vi "Planta pilot.vi"() -> ()   [LabVIEW 2022 SP3]
panel:
  out "Numeric 6":dbl
  out "Numeric 5":dbl
  out "Numeric 4":dbl
  out "Numeric 3":dbl
  out "Numeric 2":dbl
  out "Boolean":bool
  out "Numeric":dbl
  out "Presión tanque alta":dbl[](graph)
  out "Presión tanque baja":dbl[](graph)
  out "Producción de Hidrogeno":dbl[](graph)
  out "Producción Solar":dbl[](graph)
  in  "stop":bool
  # "H2"
  # "H2 baja presión"
  # "H2 alta presión"
  # "Tanc baixa pressió"
  # "barg"
  # "Tanc alta pressió"
  # "Electrolizador"
  # "Compresor"
  # "kg/h"
  # "barg"
  # "Solar"
  # "Fuel Cell"
  # "kW"
  # "kg"
  # "kW"
  # "Xarxa electrica"
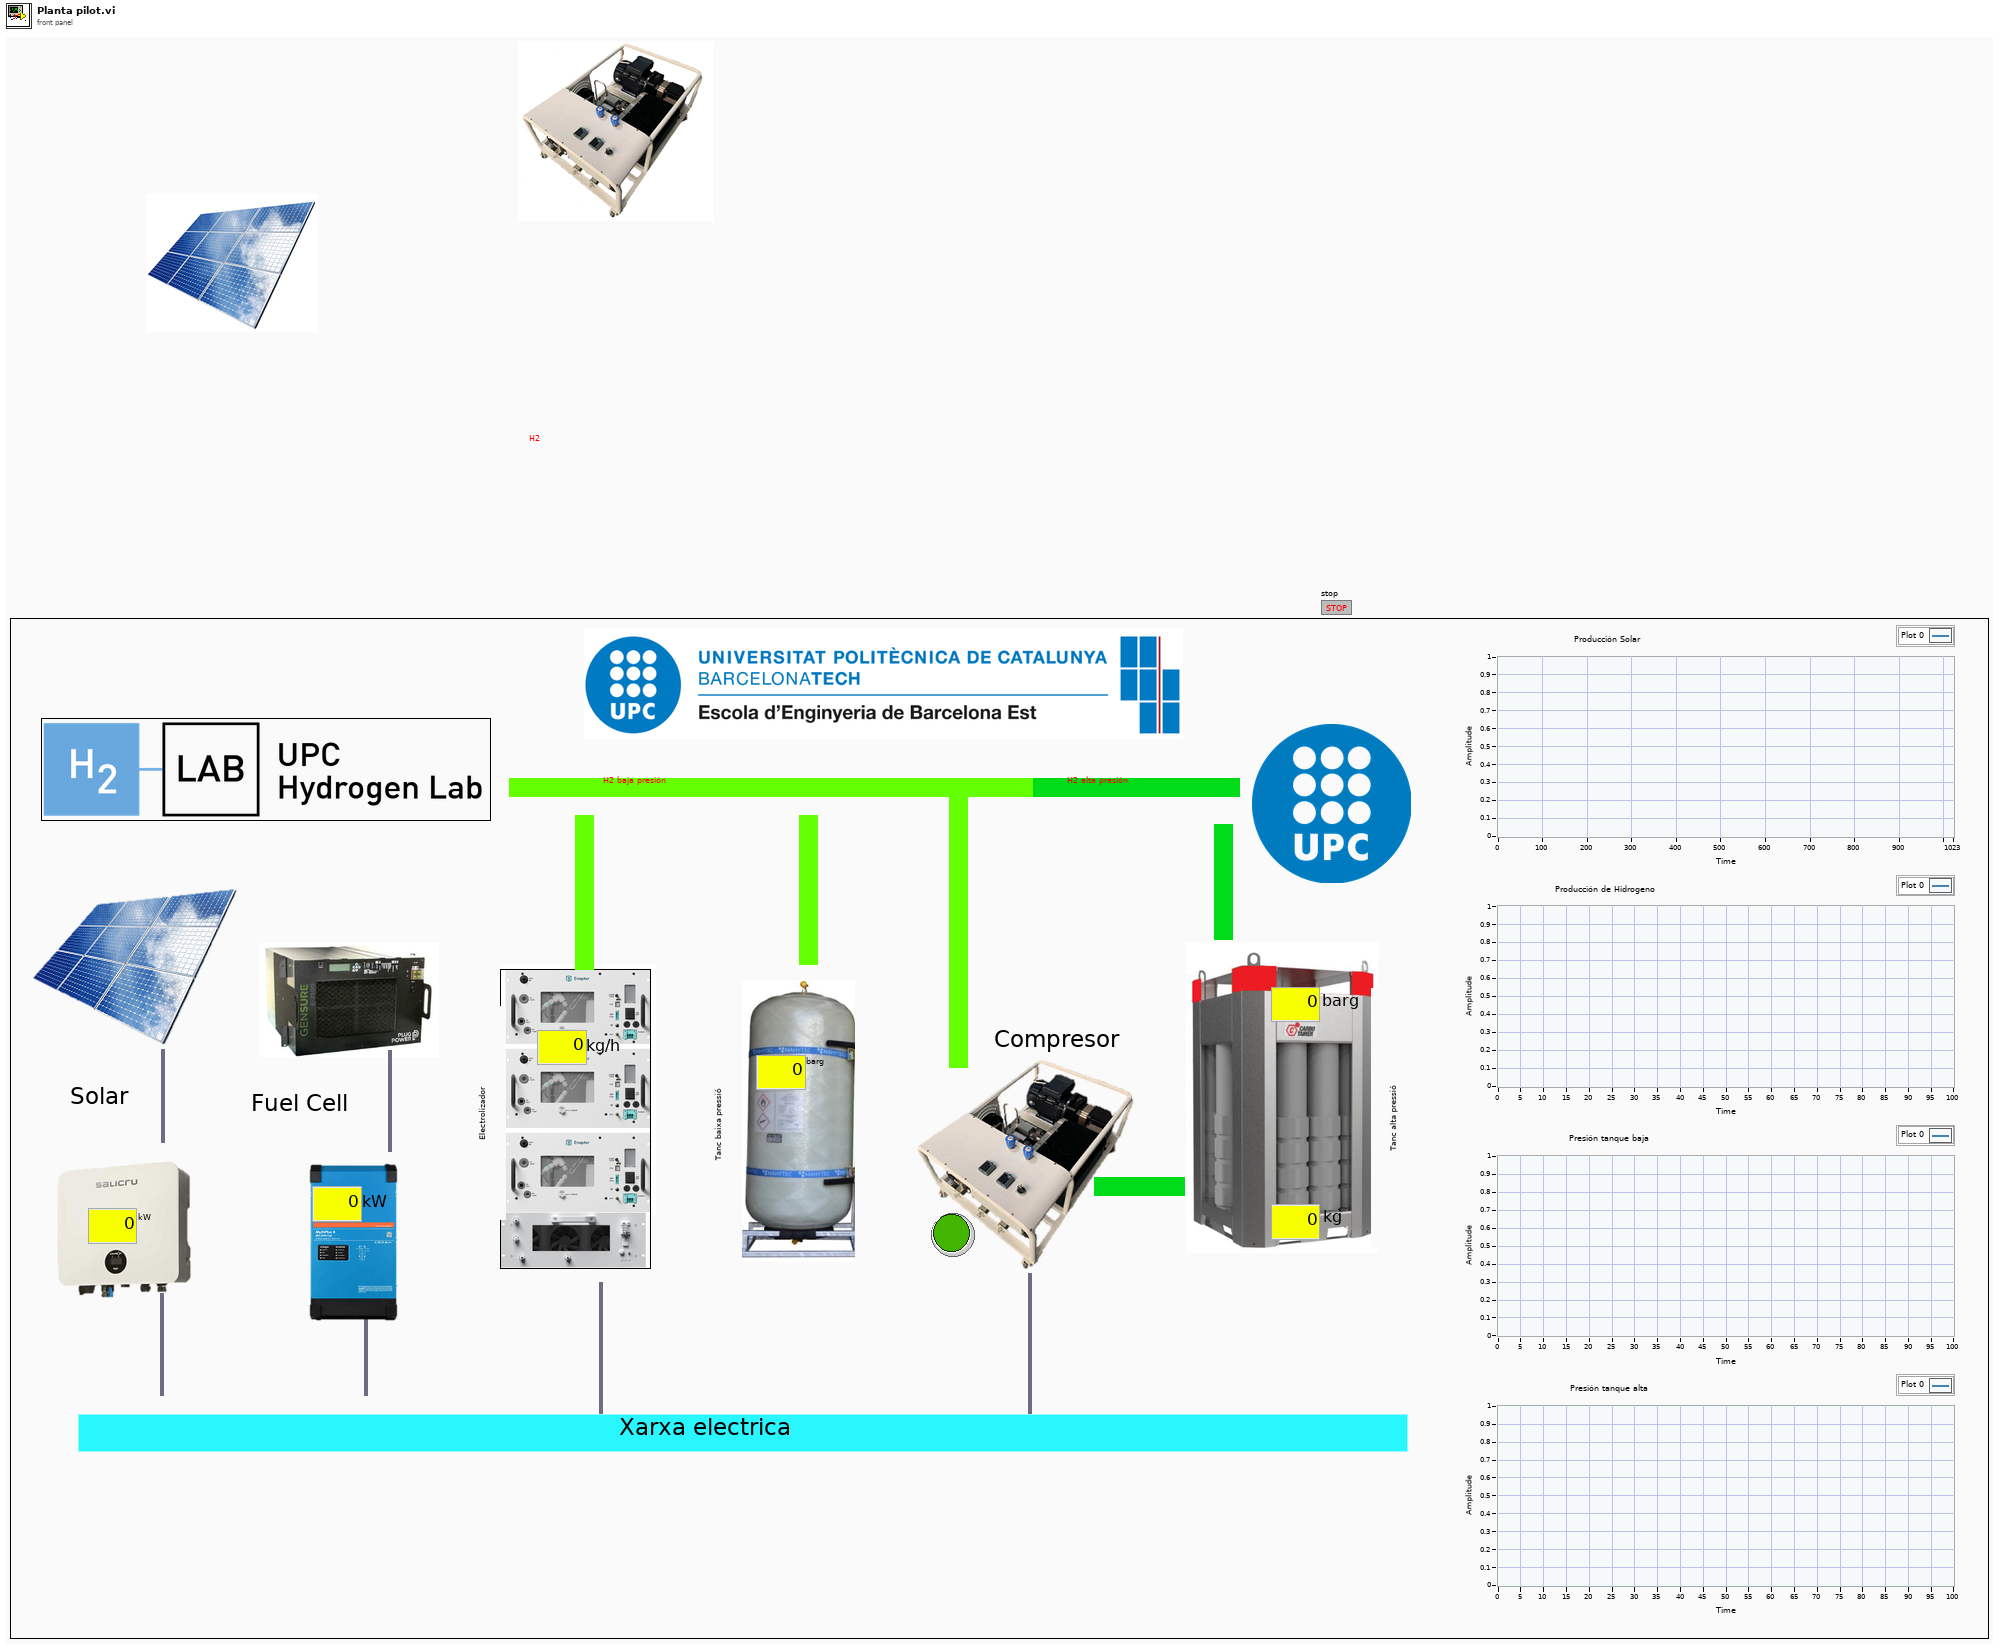
[diagram p1: front panel]
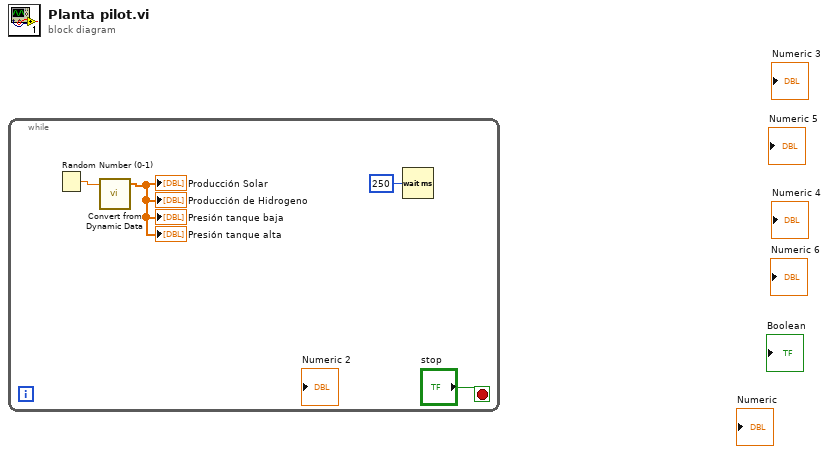
[diagram p0: block diagram]
diagram:
  n1 = while {
    stop <- "stop" stop-if-true
    n2 = Random Number (0-1)() -> (number: 0 to 1=w3:dbl)
    n3 = call "Convert from Dynamic Data"("Dynamic Data Type"=w3) -> ("Array"=→"Producción Solar" →"Producción de Hidrogeno" →"Presión tanque baja" →"Presión tanque alta":dbl[])  [unwired: 3 in]
    n4 = Wait (ms)(milliseconds to wait=u32 250) -> ()  [unwired: 1 out]
  }
